vi "analyzeImage.vi"(5 "Reinitialize position":bool, 7 "error in":errorcluster, 8 "Height":u32, 9 "Width":u32, 10 "Input cluster":T1) -> (0 "error out":errorcluster, 1 "Cars found":i32, 2 "Image out":T5(plugin-control), 3 "Output cluster":T1, 4 "Distance":sgl(graph))   [LabVIEW 2020]
doc: "Analyze image with a neural network, filter results and return calculated distance"
uses:
  controls/StateMachineVariables.ctl
  <vilib>/vision/Avi.llb/IMAQ AVI2 Refnum.ctl
  <vilib>/userDefined/High Color/IMAQdx.ctl
  <vilib>/vision/Deep Learning.llb/IMAQ DL Model Refnum.ctl
  <vilib>/vision/Image Controls.llb/IMAQ Image.ctl
  <vilib>/vision/Deep Learning.llb/IMAQ DL Model Detect Objects Node Names.ctl
  <vilib>/vision/Deep Learning.llb/IMAQ DL Model Label.ctl
  <vilib>/vision/NI_Vision_Development_Module.lvlib
panel:
  out "Relative speed":sgl(graph)
  out "Car found":bool
  in  "Minimum Score Threshold":sgl=0.3 min=0 max=1 step=0.1 format="%.3g"
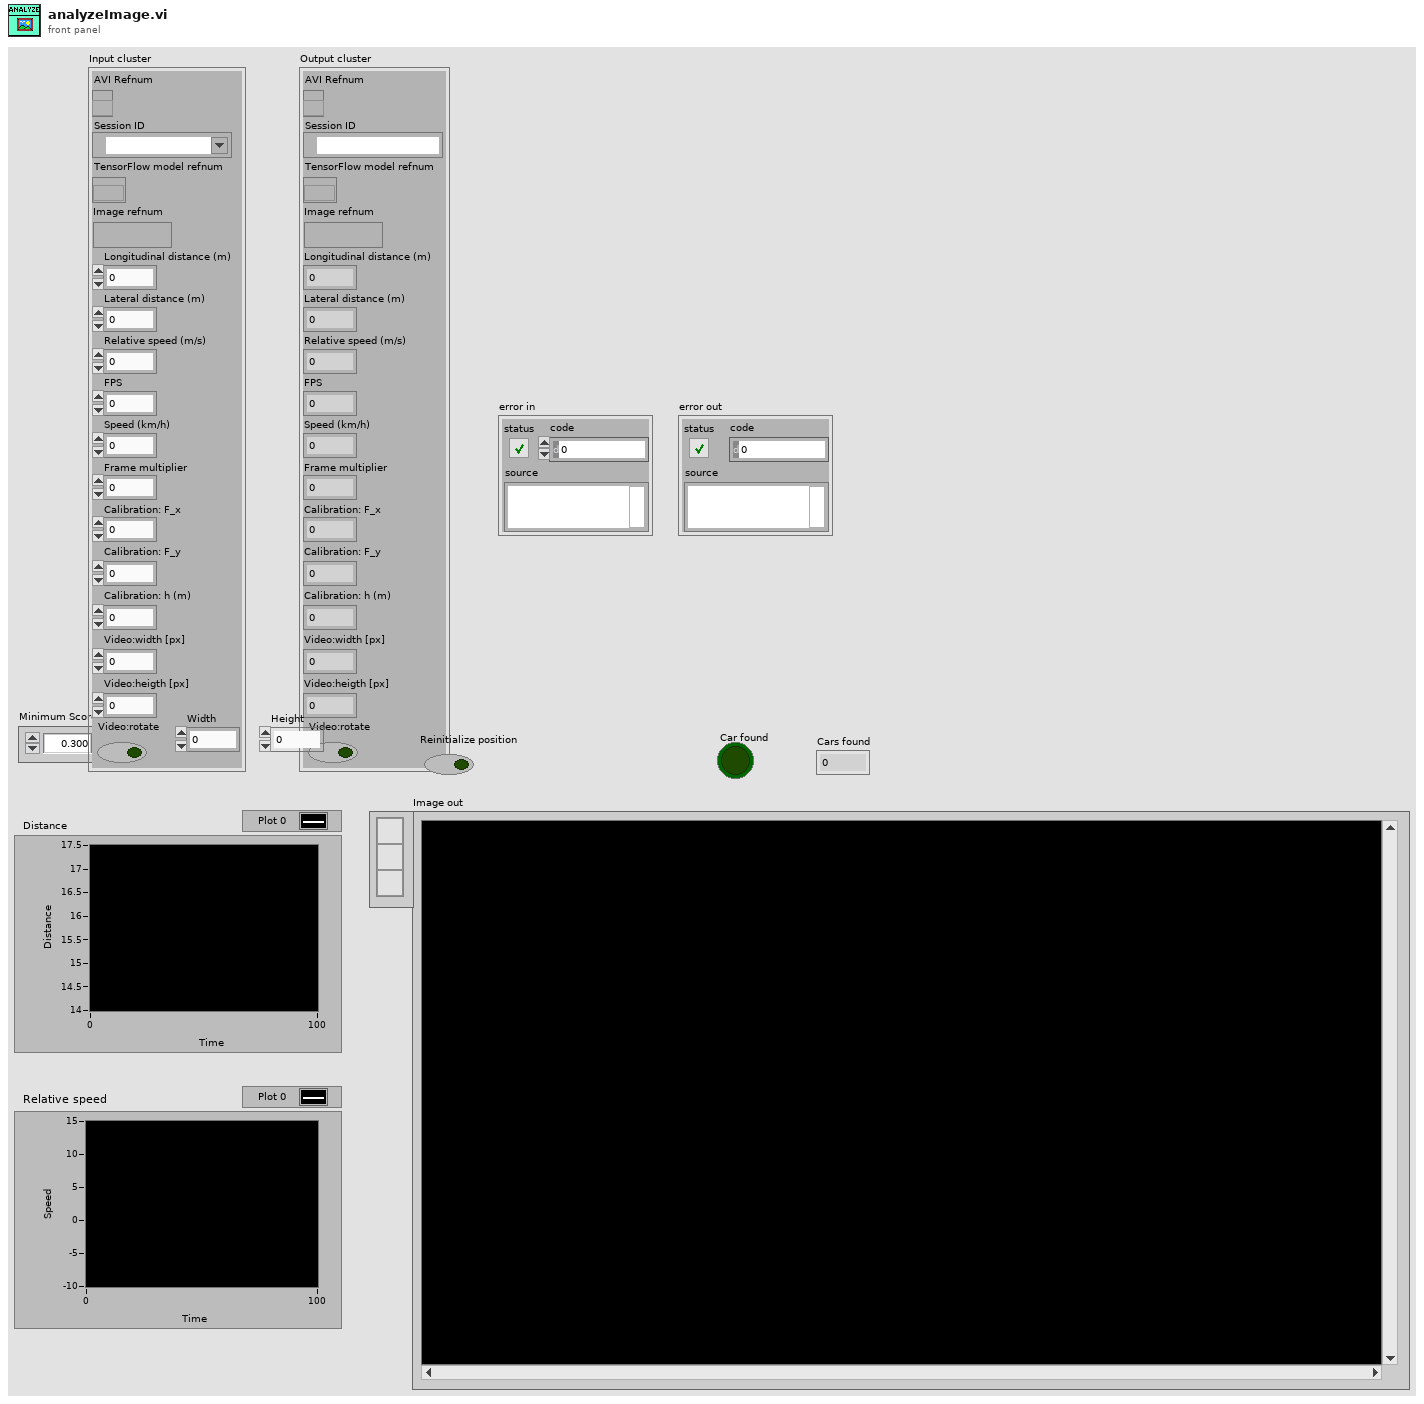
[diagram p1: front panel]
types:
  T1 = typedef "StateMachineVariables.ctl" = cluster{"AVI Refnum":T2, "Session ID":T3, "TensorFlow model refnum":T4, "Image refnum":T5, "Longitudinal distance (m)":dbl, "Lateral distance (m)":dbl, "Relative speed (m/s)":dbl, "FPS":dbl, "Speed (km/h)":dbl, "Frame multiplier":u32, "Calibration: F_x":dbl, "Calibration: F_y":dbl, "Calibration: h (m)":dbl, "Video:width [px]":i32, "Video:heigth [px]":i32, "Video:rotate":bool}
  T2 = typedef "IMAQ AVI2 Refnum.ctl" = refnum<k20>
  T3 = typedef "IMAQdx.ctl" = refnum<k21>
  T4 = typedef "IMAQ DL Model Refnum.ctl" = refnum<k20>
  T5 = typedef "IMAQ Image.ctl" = refnum<image>
  T6 = typedef "IMAQ DL Model Label.ctl" = cluster{"ID":u32, "Label":string}
  T7 = typedef "IMAQ DL Model Detect Objects Node Names.ctl" = cluster{"Number of Objects":string, "Labels":string, "Scores":string, "Bounding Boxes":string}
  T8 = typedef "IMAQ DL Model Output Data.ctl" = cluster{"Node Name":string, "Data":sgl[], "Dimensions":u64[]}
  T9 = typedef "IMAQ DL Model Objects.ctl" = cluster{"Label":string, "Score":sgl, "Bounding Box":cluster{"x":sgl, "y":sgl}[]}
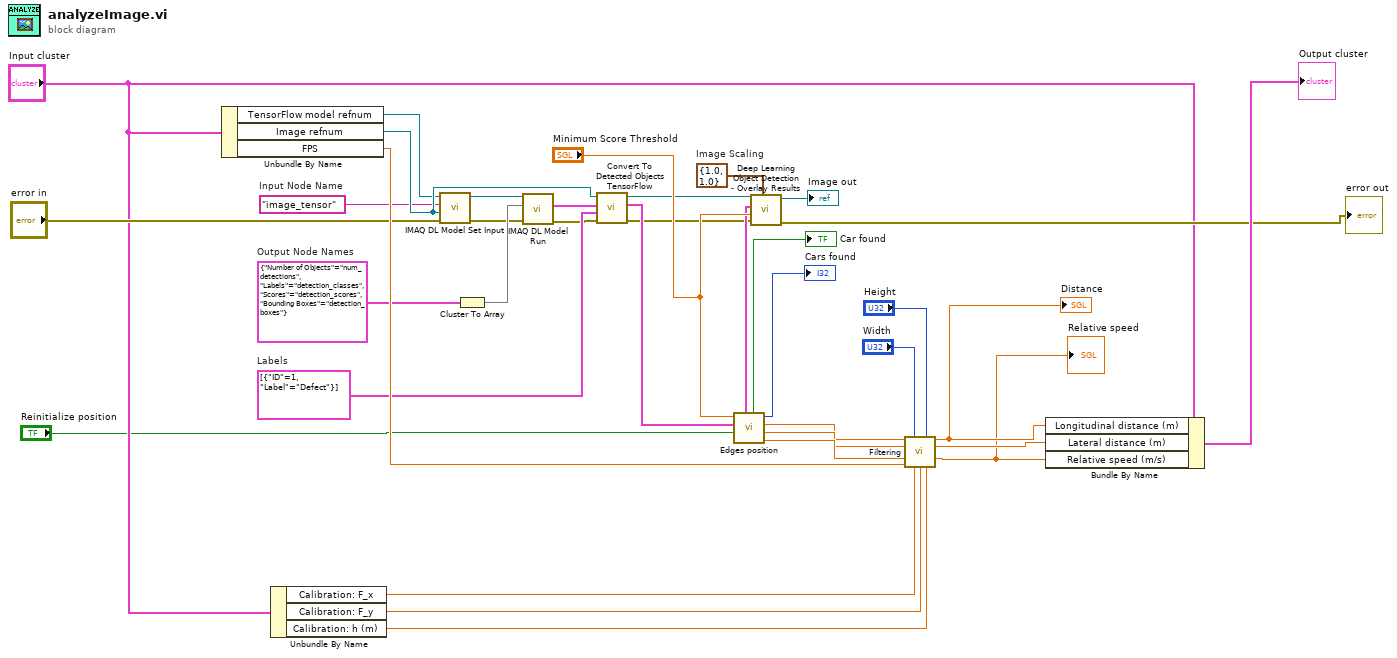
[diagram p0: block diagram]
diagram:
  w20 = T6[] [{"ID"=1, "Label"="Defect"}]  # Labels
  w18 = T7 {"Number of Objects"="num_detections", "Labels"="detection_classes", "Scores"="detection_scores", "Bounding Boxes"="detection_boxes"}  # Output Node Names
  w12 = "image_tensor"  # Input Node Name
  w11 = cluster{"X":dbl, "Y":dbl} {"X"=1.0, "Y"=1.0}  # Image Scaling
  n1 = Unbundle By Name("Input cluster") -> ("TensorFlow model refnum"=w29:T4, "Image refnum"=w33:T5, "FPS"=w35:dbl)
  n2 = Unbundle By Name("Input cluster") -> ("Calibration: F_x"=w4:dbl, "Calibration: F_y"=w3:dbl, "Calibration: h (m)"=w2:dbl)
  n3 = call-poly "IMAQ DL Model Set Input"("error in (no error)"="error in", "Image"=w33, "Input Node Name"=w12, "Model Refnum In"=w29) -> ("error out"=w14:errorcluster, "Model Refnum Out"=w13:T4)  [unwired: 5 in, 1 out]
  n4 = Cluster To Array(cluster=w18) -> (array=w19:string[])
  n5 = call "IMAQ DL Model Run"("error in (no error)"=w14, "Output Node Names"=w19, "Model Refnum In"=w13) -> ("error out"=w15:errorcluster, "Output Data Array"=w17:T8[])  [unwired: 6 in, 1 out]
  n6 = call "Convert To Detected Objects TensorFlow.vi"("error in (no error)"=w15, "Labels"=w20, "Output Data Array"=w17, "Image"=w33) -> ("error out"=w16:errorcluster, "Detected Objects"=w24:T9[], "Image (duplicate)"=w21:T5)  [unwired: 4 in, 1 out]
  n7 = call "Edges position.vi"("reinitialize position"="Reinitialize position", "Detected Objects"=w24, "Minimum Score Threshold"="Minimum Score Threshold") -> ("bottom border"=w28:sgl, "left border"=w27:sgl, "right border"=w26:sgl, "Cars found"=→"Cars found":i32, "Car found"=→"Car found":bool, "nearest car object"=w25:T9[])  [unwired: 3 in]
  n8 = call "Deep Learning Object Detection - Overlay Results.vi"("Image Scaling"=w11, "error in (no error)"=w16, "Minimum Score Threshold"="Minimum Score Threshold", "Detected Objects"=w25, "Image In"=w21) -> ("error out"=→"error out":errorcluster, "Image Out"=→"Image out":T5)  [unwired: 5 in]
  n9 = call "Filtering.vi"("Right border"=w26, "width"="Width", "height"="Height", "Left border"=w27, "Bottom border"=w28, "fps"=w35, "F_x"=w4, "F_y"=w3, "h"=w2) -> ("distance"=w31:sgl, "lateral distance"=w32:sgl, "relative speed"=w6:sgl)  [unwired: 4 in]
  "Distance" <- w31
  "Relative speed" <- w6
  n10 = Bundle By Name(cluster="Input cluster", "Longitudinal distance (m)"=w31, "Lateral distance (m)"=w32, "Relative speed (m/s)"=w6) -> (→"Output cluster":T1)
